vi "UHR-Fleezers Control (host) - 12.7d.vi"() -> ()   [LabVIEW 2012] (continued)
                    }
                  }
                  n1699 = local read "BD 2 Frequency 1 (MHz)"() -> (w2497:dbl)
                  n1700 = Select(t=w2498, s="Scan axis 2", f=w2497) -> (s? t:f=w2501:dbl)
                  n1701 = Add(x=w2489, y=w2501) -> (x+y=w2495:dbl)
                  n1702 = Select(t=w2495, s="Scan axis 2", f=w2498) -> (s? t:f=w2504:dbl)
                  n1703 = Select(t=w2497, s="Scan axis 2", f=w2495) -> (s? t:f=w2503:dbl)
                  n1704 = local read "BD 2 Frequency 2 (MHz)"() -> (w2506:dbl)
                  n1705 = local read "BD 2 Frequency 3 (MHz)"() -> (w2505:dbl)
                  n1706 = local read "Y RF Frequency Limits (MHz)"() -> (w2499:T16)
                  n1707 = local read "X RF Frequency Limits (MHz)"() -> (w2500:T16)
                  n1708 = local read "BD 1 Frequency 3 (MHz)"() -> (w2507:dbl)
                  n1709 = call "set RF board frequency - interlace.vi"("Board 2 Frequency Limits"=w2499, "Board 1 Frequency Limits"=w2500, "FPGA VI Reference In"=w2487, "Board 2 Frequency 3 (MHz)"=w2505, "Board 1 Frequency 3 (MHz)"=w2507, "Board 2 Frequency 2 (MHz)"=w2506, "Board 2 Frequency 1 (MHz)"=w2503, "Board 1 Frequency 2 (MHz)"=w2490, "Board 1 Frequency 1  (MHz)"=w2504) -> ()  [unwired: 1 in, 2 out]
                }
                frame #1 {
                  n1710 = And(x=w2558, y=w2555) -> (x .and. y?=w2557:bool)
                  n1711 = case "Only if were fishing and now formed tether" shown="True" w2557 {
                    tunnel: w2556 -> [w2560 w2575]
                    tunnel: [w2559 w2574] -> w2554
                    tunnel: w2553 -> [_ w2570]
                    frame False {
                      n1712 = local read "Fish for Tether"() -> (w2559:bool)
                      n1713 = case shown="False" w2559 {
                        tunnel: w2560 -> [w2561 _]
                        frame False {
                          n1714 = property on="BD 1 Frequency 1 (MHz)" class="DigNum (strict)"("Val(Sgnl)"=w2561) -> ()  [unwired: 2 in, 2 out]
                        }
                        frame True {
                        }
                      }
                    }
                    frame True {
                      w2574 = FALSE ("Fish for Tether")
                      n1715 = call <vilib>:"Beep.vi"() -> ()  [unwired: 3 in, 9 out]
                      n1716 = Number To Decimal String(number=w2570, width (-)=i16 1) -> (decimal integer string=w2568:string)
                      n1717 = Concatenate Strings("Formed tether in ", w2568, " attempt(s)." ("string")) -> (w2565:string)
                      n1718 = local read "Messages"() -> (w2572:string)
                      n1719 = local write "Fish for Tether"(w2574) -> ()
                      n1720 = call "Update messages.vi"("Message to add"=w2565, "Old message string"=w2572) -> ("New message string"=w2571:string)
                      n1721 = local write "Messages"(w2571) -> ()
                      n1722 = Get Date/Time In Seconds() -> (seconds since 1Jan1904=→"Time tether formed":timestamp)
                      n1723 = local read "Flow ON during cal?"() -> (w2562:bool)
                      n1724 = property on="Sample Channel\nFlow" class="Bool (strict)"("Val(Sgnl)"=w2562) -> (error out=w2563:errorcluster)  [unwired: 2 in, 1 out]
                      n1725 = case shown="\"2\", \"3\", \"4\", \"5\", \"6\"" "Then..." {
                        selector: "Then..." -> [_ w2578]
                        tunnel: w2575 -> [w2577 _]
                        tunnel: w2563 -> [_ _]
                        frame "1", Default {
                          n1726 = property on="BD 1 Frequency 1 (MHz)" class="DigNum (strict)"("Val(Sgnl)"=w2577) -> ()  [unwired: 2 in, 2 out]
                        }
                        frame "2", "3", "4", "5", "6" {
                          n1727 = flat-sequence {
                            tunnel: w2578 -> [w2580]
                            frame #0 {
                              n1728 = property on="Trap Delta (MHz)" class="DigNum (strict)"("Val(Sgnl)"="Move to Delta 1 (MHz)") -> ()  [unwired: 2 in, 2 out]
                            }
                            frame #1 {
                              n1729 = case shown="\"5\", \"6\"" w2580 {
                                selector: w2580 -> [w2583 w2593 _]
                                frame "3", "4" {
                                n1730 = flat-sequence {
                                tunnel: w2583 -> [w2584]
                                tunnel: [w2584] -> w2581
                                tunnel: [w2586] -> w2582
                                tunnel: w2581 -> [w2586]
                                tunnel: w2582 -> [w2590]
                                frame #0 {
                                n1731 = property on="Green Laser ON" class="Bool (strict)"("Val(Sgnl)"=TRUE ("Value (Signaling)")) -> ()  [unwired: 2 in, 2 out]
                                }
                                frame #1 {
                                n1732 = Multiply(x="Wait Before Save (s)", y=u32 1000 ("x")) -> (x*y=w2588:u32)
                                n1733 = Wait (ms)(milliseconds to wait=w2588) -> ()  [unwired: 1 out]
                                }
                                frame #2 {
                                n1734 = property on="Start Saving" class="Bool (strict)"("Value"=TRUE ("Start Saving")) -> ()  [unwired: 2 in, 2 out]
                                n1735 = case shown="\"4\"" w2590 {
                                frame Default {
                                }
                                frame "4" {
                                n1736 = property on="Fl. Triggered..." class="Bool (strict)"("Val(Sgnl)"=TRUE ("Value (Signaling)")) -> ()  [unwired: 2 in, 2 out]
                                }
                                }
                                }
                                }
                                }
                                frame "5", "6" {
                                n1737 = stacked-sequence {
                                tunnel: w2593 -> [_ _ _ _ _ _ w2605]
                                frame #0 {
                                n1738 = Replace Array Subset(array=u32[] [0] ("Index Values"), new element="Raster Set Upon Tether", index=0) -> (w2594:u32[])
                                n1739 = property on="Saved AOD Raster Scan Parameter Sets" class="Arr (strict)"("Index Values"=w2594) -> ()  [unwired: 2 in, 2 out]
                                }
                                frame #1 {
                                n1740 = Wait (ms)(milliseconds to wait=u32 500) -> ()  [unwired: 1 out]
                                }
                                frame #2 {
                                n1741 = property on="Load parameters" class="Bool (strict)"("Val(Sgnl)"=TRUE ("Value (Signaling)")) -> ()  [unwired: 2 in, 2 out]
                                n1742 = case shown="True" "Green ON During Raster" {
                                frame False {
                                }
                                frame True {
                                n1743 = property on="Green Laser ON" class="Bool (strict)"("Val(Sgnl)"=TRUE ("Value (Signaling)")) -> ()  [unwired: 2 in, 2 out]
                                }
                                }
                                }
                                frame #3 {
                                n1744 = Wait (ms)(milliseconds to wait=u32 500) -> ()  [unwired: 1 out]
                                }
                                frame #4 {
                                n1745 = property on="Trap Raster Scan" class="Bool (strict)"("Val(Sgnl)"=TRUE ("Value (Signaling)")) -> ()  [unwired: 2 in, 2 out]
                                }
                                frame #5 {
                                n1746 = Wait (ms)(milliseconds to wait=u32 2000) -> ()  [unwired: 1 out]
                                }
                                frame #6 {
                                n1747 = flat-sequence {
                                tunnel: w2605 -> [w2612]
                                frame #0 {
                                n1748 = while {
                                stop <- w2608 stop-if-true
                                n1749 = local read "Raster Scanning..."() -> (w2607:bool)
                                n1750 = local read "Saving..."() -> (w2610:bool)
                                n1751 = Wait (ms)(milliseconds to wait=u32 100) -> ()  [unwired: 1 out]
                                n1752 = Not(x=w2610) -> (.not. x?=w2609:bool)
                                n1753 = Not(x=w2607) -> (.not. x?=w2606:bool)
                                n1754 = And(x=w2609, y=w2606) -> (x .and. y?=w2608:bool)
                                }
                                }
                                frame #1 {
                                n1755 = local read "Tether"() -> (w2613:bool)
                                n1756 = case shown="True" w2613 {
                                tunnel: w2612 -> [_ w2615]
                                frame False {
                                n1757 = property on="Fish for Tether" class="Bool (strict)"("Val(Sgnl)"="Fish again after \nraster break?") -> ()  [unwired: 2 in, 2 out]
                                }
                                frame True {
                                n1758 = stacked-sequence {
                                tunnel: w2615 -> [_ w2619 _ _]
                                frame #0 {
                                n1759 = property on="Trap Delta (MHz)" class="DigNum (strict)"("Val(Sgnl)"="Move to Delta 2 (MHz)") -> ()  [unwired: 2 in, 2 out]
                                n1760 = case shown="True" "Flow ON after\ntether testing?" {
                                frame False {
                                }
                                frame True {
                                n1761 = property on="Sample Channel\nFlow" class="Bool (strict)"("Val(Sgnl)"=TRUE ("Value (Signaling)")) -> ()  [unwired: 2 in, 2 out]
                                }
                                }
                                }
                                frame #1 {
                                n1762 = flat-sequence {
                                tunnel: w2619 -> [w2621]
                                frame #0 {
                                n1763 = Wait (ms)(milliseconds to wait=u32 500) -> ()  [unwired: 1 out]
                                }
                                frame #1 {
                                n1764 = case shown="\"6\"" w2621 {
                                frame Default {
                                }
                                frame "6" {
                                n1765 = property on="Green Laser ON" class="Bool (strict)"("Val(Sgnl)"=TRUE ("Green Laser ON/Interlacing")) -> ()  [unwired: 2 in, 2 out]
                                }
                                }
                                }
                                frame #2 {
                                n1766 = Wait (ms)(milliseconds to wait=u32 500) -> ()  [unwired: 1 out]
                                }
                                frame #3 {
                                n1767 = local write "Start Saving"("Save at end (5, 6)") -> ()
                                }
                                }
                                }
                                frame #2 {
                                n1768 = local read "Bead Sep. Int. Time (s)"() -> (w2627:dbl)
                                n1769 = Multiply(x=w2627, y=1000.0) -> (x*y=w2626:dbl)
                                n1770 = Wait (ms)(milliseconds to wait=w2626) -> ()  [unwired: 1 out]
                                }
                                frame #3 {
                                n1771 = property on="Remove Offset" class="Bool (strict)"("Val(Sgnl)"=TRUE ("Value (Signaling)")) -> ()  [unwired: 2 in, 2 out]
                                }
                                }
                                }
                                }
                                }
                                }
                                }
                                }
                                }
                                frame "2", Default {
                                }
                              }
                            }
                          }
                        }
                      }
                      "Tether" <- "Tether Alarm?"
                    }
                  }
                }
                frame #2 {
                  n1772 = local read "Oscillate Set 1"() -> (w2634:bool)
                  n1773 = local read "Stop All"() -> (w2632:bool)
                  n1774 = Or(x=w2634, y=w2629) -> (x .or. y?=w2631:bool)
                  n1775 = Not(x=w2631) -> (.not. x?=w2633:bool)
                  n1776 = Compound Arithmetic op=OR(w2632, w2633) -> (w2630:bool)
                }
              }
              n1777 = node-c288() -> ()  [unwired: 2 out]
            }
            n1778 = node-c288(w2466) -> ()  [unwired: 1 out]
          }
        }
      }
      event "Fl. Triggered...": Value Change {
        n1779 = event-data() -> ()  [unwired: 7 out]
        n1780 = case shown="True" "Fl. Triggered..." {
          frame False {
          }
          frame True {
            n1781 = node-c288() -> (w2645:T23)  [unwired: 4 out]
            n1782 = timed-loop {
              timing: w2645 -> [_]
              timing-out: [_] -> w2644
              tunnel: "Action" -> [w2653]
              shift-right: [w2650] -> _
              shift-left: u8 255 -> [w2652]
              shift-right: [w2647] -> _
              shift-left: 255 -> [w2649]
              stop <- w2646 stop-if-true
              # "Reset confocal spot"
              n1783 = node-c288() -> ()  [unwired: 2 out]
              n1784 = flat-sequence {
                tunnel: w2653 -> [w2673]
                tunnel: w2652 -> [w2672]
                tunnel: [w2671] -> w2651
                tunnel: w2649 -> [w2658]
                tunnel: [w2657] -> w2648
                tunnel: [w3052] -> w2646
                tunnel: w2651 -> [w3051]
                tunnel: [w3051] -> w2650
                tunnel: [w3050] -> w2647
                tunnel: w2648 -> [w3050]
                frame #0 {
                  n1785 = local read "Delta Fl. 2"() -> (w2670:dbl)
                  n1786 = local read "Delta Fl. 1"() -> (w2665:dbl)
                  n1787 = Multiply(x="Fl. Delta Thresh. (kHz)", y=1000.0) -> (x*y=w2660:dbl)
                  n1788 = Select(t=w2665, s="APD to Watch", f=w2670) -> (s? t:f=w2661:dbl)
                  n1789 = Greater?(x=w2661, y=w2660) -> (0:w2666:bool)
                  n1790 = Or(x="Force Yank", y=w2666) -> (x .or. y?=w2664:bool)
                  n1791 = And(x=w2664, y="Yank when?") -> (x .and. y?=w2662:bool)
                  n1792 = case shown="False" w2662 {
                    tunnel: w2673 -> [w2676 w2877]
                    tunnel: w2672 -> [w2678 w2873]
                    tunnel: [w2678 w2871] -> w2671
                    tunnel: w2661 -> [w2684 _]
                    tunnel: w2660 -> [w2683 _]
                    tunnel: "Force Yank" -> [w2681 _]
                    tunnel: w2658 -> [w2680 w2870]
                    tunnel: [w2679 w2870] -> w2657
                    frame False {
                      n1793 = Negate(x=w2683) -> (-x=w2675:dbl)
                      n1794 = local write "Fl. High"(TRUE ("Fl. High")) -> ()
                      n1795 = Less?(x=w2684, y=w2675) -> (x < y?=w2682:bool)
                      n1796 = Or(x=w2681, y=w2682) -> (x .or. y?=w2677:bool)
                      n1797 = case shown="True" w2677 {
                        tunnel: w2680 -> [w2685 w2695]
                        tunnel: [w2685 w2694] -> w2679
                        tunnel: w2676 -> [_ w2693]
                        frame False {
                        }
                        frame True {
                          n1798 = flat-sequence {
                            tunnel: w2695 -> [w2701]
                            tunnel: w2693 -> [w2698]
                            tunnel: [w2700] -> w2692
                            tunnel: [w2699] -> w2691
                            tunnel: [w2698] -> w2690
                            tunnel: w2689 -> [w2697]
                            tunnel: [w2697] -> w2688
                            tunnel: w2687 -> [w2696]
                            tunnel: [w2696] -> w2686
                            tunnel: [w2772] -> w2694
                            tunnel: w2692 -> [w2772]
                            tunnel: w2691 -> [w2771]
                            tunnel: w2690 -> [w2770]
                            tunnel: w2688 -> [w2769]
                            tunnel: w2686 -> [w2768]
                            frame #0 {
                              n1799 = call <vilib>:"Beep.vi"() -> ()  [unwired: 12 in]
                              n1800 = local write "Waiting"(FALSE ("Waiting")) -> ()
                              n1801 = Increment(x=w2701) -> (x+1=w2700:i32)
                              n1802 = case shown="\"Image\"" w2698 {
                                tunnel: w2700 -> [_ w2706 _]
                                frame "Alarm", Default {
                                }
                                frame "Yank" {
                                n1803 = flat-sequence {
                                tunnel: w2706 -> [w2709]
                                tunnel: [w2708] -> w2705
                                tunnel: [w2707] -> w2704
                                tunnel: w2705 -> [w2719]
                                tunnel: w2704 -> [w2720]
                                frame #0 {
                                n1804 = local read "Yank Delay (s)"() -> (w2712:dbl)
                                n1805 = local read "N Array El"() -> (w2707:u8)
                                n1806 = Quotient & Remainder(x=w2709, y=w2707) -> (x-y*floor(x/y)=w2708:i32)  [unwired: 1 out]
                                n1807 = Multiply(x=w2712, y=1000.0) -> (x*y=w2710:dbl)
                                n1808 = Wait (ms)(milliseconds to wait=w2710) -> ()  [unwired: 1 out]
                                }
                                frame #1 {
                                n1809 = local read "Yank to which?"() -> (w2714:bool)
                                n1810 = local read "Random Choice"() -> (w2724:bool)
                                n1811 = local read "Yank to Trap Delta (MHz)"() -> (w2717:dbl[])
                                n1812 = local read "Yank to SP"() -> (w2718:dbl[])
                                n1813 = Random Number (0-1)() -> (number: 0 to 1=w2723:dbl)
                                n1814 = Multiply(x=w2720, y=w2723) -> (x*y=w2722:dbl)
                                n1815 = Round Toward -Infinity(1:w2722) -> (0:w2721:dbl)
                                n1816 = Select(t=w2721, s=w2724, f=w2719) -> (s? t:f=w2715:dbl)
                                n1817 = Select(t=w2717, s=w2714, f=w2718) -> (s? t:f=w2716:dbl[])
                                n1818 = Index Array(array=w2716, index=w2715) -> (element=w2713:dbl)
                                n1819 = case shown="True" w2714 {
                                tunnel: w2713 -> [w2725 w2752]
                                frame False {
                                n1820 = flat-sequence {
                                tunnel: w2725 -> [w2726]
                                frame #0 {
                                n1821 = property on="Trap Pos FB SP" class="DigNum (strict)"("Val(Sgnl)"=w2726) -> ()  [unwired: 2 in, 2 out]
                                }
                                frame #1 {
                                n1822 = Wait (ms)(milliseconds to wait=u32 700) -> ()  [unwired: 1 out]
                                }
                                frame #2 {
                                n1823 = local read "Action (%)"() -> (w2731:dbl)
                                n1824 = Absolute Value(x=w2731) -> (abs(x)=w2730:dbl)
                                n1825 = Greater?(x=w2730, y=70.0) -> (0:w2728:bool)
                                n1826 = property on="Remove Action Offset" class="Bool (strict)"("Val(Sgnl)"=w2728) -> ()  [unwired: 2 in, 2 out]
                                }
                                frame #3 {
                                n1827 = for {
                                N: 4 -> [_]
                                n1828 = flat-sequence {
                                frame #0 {
                                n1829 = Wait (ms)(milliseconds to wait=u32 500) -> ()  [unwired: 1 out]
                                }
                                frame #1 {
                                n1830 = local read "Action (%)"() -> (w2737:dbl)
                                n1831 = Absolute Value(x=w2737) -> (abs(x)=w2736:dbl)
                                n1832 = Greater?(x=w2736, y=70.0) -> (0:w2734:bool)
                                n1833 = property on="Remove Action Offset" class="Bool (strict)"("Val(Sgnl)"=w2734) -> ()  [unwired: 2 in, 2 out]
                                }
                                }
                                }
                                }
                                frame #4 {
                                n1834 = Wait (ms)(milliseconds to wait=u32 500) -> ()  [unwired: 1 out]
                                }
                                frame #5 {
                                n1835 = local read "Mean"() -> (w2745:dbl)
                                n1836 = Greater?(x=w2745, y=11.0) -> (0:w2739:bool)
                                n1837 = Not(x=w2739) -> (.not. x?=w2740:bool)
                                n1838 = And(x=w2740, y="Shift confocal") -> (x .and. y?=w2742:bool)
                                n1839 = And(x=w2739, y="Shift confocal") -> (x .and. y?=w2743:bool)
                                n1840 = case shown="True" w2743 {
                                frame False {
                                }
                                frame True {
                                n1841 = local read "Confocal Y 2 (V)"() -> (w2749:dbl)
                                n1842 = local read "Confocal X 2 (V)"() -> (w2748:dbl)
                                n1843 = property on="AO1" class="Slide (strict)"("Val(Sgnl)"=w2749) -> ()  [unwired: 2 in, 2 out]
                                n1844 = property on="AO2" class="Slide (strict)"("Val(Sgnl)"=w2748) -> ()  [unwired: 2 in, 2 out]
                                }
                                }
                                n1845 = case shown="True" w2742 {
                                frame False {
                                }
                                frame True {
                                n1846 = local read "Confocal Y 1 (V)"() -> (w2747:dbl)
                                n1847 = local read "Confocal X 1 (V)"() -> (w2746:dbl)
                                n1848 = property on="AO1" class="Slide (strict)"("Val(Sgnl)"=w2747) -> ()  [unwired: 2 in, 2 out]
                                n1849 = property on="AO2" class="Slide (strict)"("Val(Sgnl)"=w2746) -> ()  [unwired: 2 in, 2 out]
                                }
                                }
                                }
                                frame #6 {
                                n1850 = Wait (ms)(milliseconds to wait=u32 1500) -> ()  [unwired: 1 out]
                                }
                                frame #7 {
                                n1851 = property on="Rem fb disp offset" class="Bool (strict)"("Val(Sgnl)"=TRUE ("Value (Signaling)")) -> ()  [unwired: 2 in, 2 out]
                                }
                                }
                                }
                                frame True {
                                n1852 = flat-sequence {
                                tunnel: w2752 -> [w2753]
                                frame #0 {
                                n1853 = property on="Trap Delta (MHz)" class="DigNum (strict)"("Val(Sgnl)"=w2753) -> ()  [unwired: 2 in, 2 out]
                                }
                                frame #1 {
                                n1854 = Wait (ms)(milliseconds to wait=u32 500) -> ()  [unwired: 1 out]
                                }
                                frame #2 {
                                n1855 = local read "Shift confocal"() -> (w2759:bool)
                                n1856 = local read "Mean"() -> (w2761:dbl)
                                n1857 = Greater?(x=w2761, y=11.0) -> (0:w2758:bool)
                                n1858 = Not(x=w2758) -> (.not. x?=w2757:bool)
                                n1859 = And(x=w2757, y=w2759) -> (x .and. y?=w2755:bool)
                                n1860 = And(x=w2758, y=w2759) -> (x .and. y?=w2756:bool)
                                n1861 = case shown="True" w2756 {
                                frame False {
                                }
                                frame True {
                                n1862 = local read "Confocal Y 2 (V)"() -> (w2765:dbl)
                                n1863 = local read "Confocal X 2 (V)"() -> (w2764:dbl)
                                n1864 = property on="AO2" class="Slide (strict)"("Val(Sgnl)"=w2764) -> ()  [unwired: 2 in, 2 out]
                                n1865 = property on="AO1" class="Slide (strict)"("Val(Sgnl)"=w2765) -> ()  [unwired: 2 in, 2 out]
                                }
                                }
                                n1866 = case shown="True" w2755 {
                                frame False {
                                }
                                frame True {
                                n1867 = local read "Confocal X 1 (V)"() -> (w2762:dbl)
                                n1868 = local read "Confocal Y 1 (V)"() -> (w2763:dbl)
                                n1869 = property on="AO2" class="Slide (strict)"("Val(Sgnl)"=w2762) -> ()  [unwired: 2 in, 2 out]
                                n1870 = property on="AO1" class="Slide (strict)"("Val(Sgnl)"=w2763) -> ()  [unwired: 2 in, 2 out]
                                }
                                }
                                }
                                }
                                }
                                }
                                }
                                }
                                }
                                frame "Image" {
                                n1871 = property on="Confocal Image" class="Bool (strict)"("Val(Sgnl)"=TRUE ("Value (Signaling)")) -> ()  [unwired: 2 in, 2 out]
                                }
                              }
                              n1872 = local write "Fl. High"(FALSE ("Fl. High")) -> ()
                              n1873 = local read "Time (s)"() -> (w2699:dbl)
                            }
                            frame #1 {
                              n1874 = case shown="True" "Auto F Reset" {
                                tunnel: w2771 -> [_ w2776]
                                tunnel: w2770 -> [_ w2775]
                                tunnel: w2769 -> [_ w2774]
                                tunnel: w2768 -> [_ w2773]
                                frame False {
                                }
                                frame True {
                                n1875 = node-c288() -> (w2778:T23)  [unwired: 4 in]
                                n1876 = timed-loop {
                                timing: w2778 -> [_]
                                timing-out: [_] -> w2777
                                tunnel: w2776 -> [w2783]
                                tunnel: w2775 -> [w2782]
                                tunnel: w2774 -> [w2781]
                                tunnel: w2773 -> [w2780]
                                stop <- w2779 stop-if-true
                                n1877 = node-c288() -> ()  [unwired: 1 in, 1 out]
                                n1878 = local read "Fl. Delta Thresh. (kHz)"() -> (w2792:dbl)
                                n1879 = local read "APD to Watch"() -> (w2793:bool)
                                n1880 = local read "Delta Fl. 1"() -> (w2794:dbl)
                                n1881 = local read "Delta Fl. 2"() -> (w2795:dbl)
                                n1882 = local read "Fl. Triggered..."() -> (w2786:bool)
                                n1883 = local read "Stop All"() -> (w2787:bool)
                                n1884 = local read "Reset Force"() -> (w2785:bool)
                                n1885 = Multiply(x=w2792, y=1000.0) -> (x*y=w2790:dbl)
                                n1886 = Select(t=w2794, s=w2793, f=w2795) -> (s? t:f=w2789:dbl)
                                n1887 = Not(x=w2786) -> (.not. x?=w2784:bool)
                                n1888 = Greater?(x=w2789, y=w2790) -> (0:w2788:bool)
                                n1889 = Compound Arithmetic op=OR(w2788, w2787, w2784, w2785) -> (w2779:bool)
                                n1890 = case shown="True" w2779 {
                                tunnel: w2783 -> [_ w2799]
                                tunnel: w2782 -> [_ w2803]
                                tunnel: w2781 -> [_ w2802]
                                tunnel: w2780 -> [_ w2801]
                                frame False {
                                }
                                frame True {
                                n1891 = case shown="\"Yank\"" w2803 {
                                tunnel: w2802 -> [_ w2813]
                                tunnel: w2801 -> [_ w2811]
                                frame "Image", Default {
                                }
                                frame "Yank" {
                                n1892 = flat-sequence {
                                tunnel: [w2816] -> w2814
                                tunnel: w2813 -> [w2816]
                                tunnel: [w2815] -> w2812
                                tunnel: w2811 -> [w2815]
                                tunnel: w2814 -> [w2822]
                                tunnel: w2812 -> [w2820]
                                frame #0 {
                                n1893 = local read "Yank Delay (s)"() -> (w2819:dbl)
                                n1894 = Multiply(x=w2819, y=1000.0) -> (x*y=w2817:dbl)
                                n1895 = Wait (ms)(milliseconds to wait=w2817) -> ()  [unwired: 1 out]
                                }
                                frame #1 {
                                n1896 = local read "Yank to which?"() -> (w2821:bool)
                                n1897 = case shown="False" w2821 {
                                tunnel: w2822 -> [_ w2850]
                                tunnel: w2820 -> [w2823 _]
                                frame False {
                                n1898 = flat-sequence {
                                tunnel: w2823 -> [w2824]
                                frame #0 {
                                n1899 = property on="Trap Pos FB SP" class="DigNum (strict)"("Val(Sgnl)"=w2824) -> ()  [unwired: 2 in, 2 out]
                                }
                                frame #1 {
                                n1900 = Wait (ms)(milliseconds to wait=u32 700) -> ()  [unwired: 1 out]
                                }
                                frame #2 {
                                n1901 = local read "Action (%)"() -> (w2829:dbl)
                                n1902 = Absolute Value(x=w2829) -> (abs(x)=w2828:dbl)
                                n1903 = Greater?(x=w2828, y=70.0) -> (0:w2826:bool)
                                n1904 = property on="Remove Action Offset" class="Bool (strict)"("Val(Sgnl)"=w2826) -> ()  [unwired: 2 in, 2 out]
                                }
                                frame #3 {
                                n1905 = for {
                                N: 4 -> [_]
                                n1906 = flat-sequence {
                                frame #0 {
                                n1907 = Wait (ms)(milliseconds to wait=u32 500) -> ()  [unwired: 1 out]
                                }
                                frame #1 {
                                n1908 = local read "Action (%)"() -> (w2835:dbl)
                                n1909 = Absolute Value(x=w2835) -> (abs(x)=w2834:dbl)
                                n1910 = Greater?(x=w2834, y=70.0) -> (0:w2832:bool)
                                n1911 = property on="Remove Action Offset" class="Bool (strict)"("Val(Sgnl)"=w2832) -> ()  [unwired: 2 in, 2 out]
                                }
                                }
                                }
                                }
                                frame #4 {
                                n1912 = Wait (ms)(milliseconds to wait=u32 500) -> ()  [unwired: 1 out]
                                }
                                frame #5 {
                                n1913 = local read "Shift confocal"() -> (w2840:bool)
                                n1914 = local read "Mean"() -> (w2843:dbl)
                                n1915 = Greater?(x=w2843, y=11.0) -> (0:w2839:bool)
                                n1916 = Not(x=w2839) -> (.not. x?=w2838:bool)
                                n1917 = And(x=w2839, y=w2840) -> (x .and. y?=w2841:bool)
                                n1918 = And(x=w2838, y=w2840) -> (x .and. y?=w2837:bool)
                                n1919 = case shown="True" w2841 {
                                frame False {
                                }
                                frame True {
                                n1920 = local read "Confocal X 2 (V)"() -> (w2846:dbl)
                                n1921 = local read "Confocal Y 2 (V)"() -> (w2847:dbl)
                                n1922 = property on="AO2" class="Slide (strict)"("Val(Sgnl)"=w2846) -> ()  [unwired: 2 in, 2 out]
                                n1923 = property on="AO1" class="Slide (strict)"("Val(Sgnl)"=w2847) -> ()  [unwired: 2 in, 2 out]
                                }
                                }
                                n1924 = case shown="True" w2837 {
                                frame False {
                                }
                                frame True {
                                n1925 = local read "Confocal Y 1 (V)"() -> (w2845:dbl)
                                n1926 = local read "Confocal X 1 (V)"() -> (w2844:dbl)
                                n1927 = property on="AO1" class="Slide (strict)"("Val(Sgnl)"=w2845) -> ()  [unwired: 2 in, 2 out]
                                n1928 = property on="AO2" class="Slide (strict)"("Val(Sgnl)"=w2844) -> ()  [unwired: 2 in, 2 out]
                                }
                                }
                                }
                                frame #6 {
                                n1929 = Wait (ms)(milliseconds to wait=u32 1500) -> ()  [unwired: 1 out]
                                }
                                frame #7 {
                                n1930 = property on="Rem fb disp offset" class="Bool (strict)"("Val(Sgnl)"=TRUE ("Value (Signaling)")) -> ()  [unwired: 2 in, 2 out]
                                }
                                }
                                }
                                frame True {
                                n1931 = flat-sequence {
                                tunnel: w2850 -> [w2851]
                                frame #0 {
                                n1932 = property on="Trap Delta (MHz)" class="DigNum (strict)"("Val(Sgnl)"=w2851) -> ()  [unwired: 2 in, 2 out]
                                }
                                frame #1 {
                                n1933 = Wait (ms)(milliseconds to wait=u32 500) -> ()  [unwired: 1 out]
                                }
                                frame #2 {
                                n1934 = local read "Shift confocal"() -> (w2857:bool)
                                n1935 = local read "Mean"() -> (w2858:dbl)
                                n1936 = Greater?(x=w2858, y=11.0) -> (0:w2856:bool)
                                n1937 = And(x=w2856, y=w2857) -> (x .and. y?=w2854:bool)
                                n1938 = Not(x=w2856) -> (.not. x?=w2855:bool)
                                n1939 = And(x=w2855, y=w2857) -> (x .and. y?=w2853:bool)
                                n1940 = case shown="True" w2854 {
                                frame False {
                                }
                                frame True {
                                n1941 = local read "Confocal Y 2 (V)"() -> (w2863:dbl)
                                n1942 = local read "Confocal X 2 (V)"() -> (w2862:dbl)
                                n1943 = property on="AO1" class="Slide (strict)"("Val(Sgnl)"=w2863) -> ()  [unwired: 2 in, 2 out]
                                n1944 = property on="AO2" class="Slide (strict)"("Val(Sgnl)"=w2862) -> ()  [unwired: 2 in, 2 out]
                                }
                                }
                                n1945 = case shown="True" w2853 {
                                frame False {
                                }
                                frame True {
                                n1946 = local read "Confocal Y 1 (V)"() -> (w2861:dbl)
                                n1947 = local read "Confocal X 1 (V)"() -> (w2860:dbl)
                                n1948 = property on="AO2" class="Slide (strict)"("Val(Sgnl)"=w2860) -> ()  [unwired: 2 in, 2 out]
                                n1949 = property on="AO1" class="Slide (strict)"("Val(Sgnl)"=w2861) -> ()  [unwired: 2 in, 2 out]
                                }
                                }
                                }
                                }
                                }
                                }
                                }
                                }
                                }
                                }
                                n1950 = local read "Time (s)"() -> (w2798:dbl)
                                n1951 = Subtract(x=w2799, y=w2798) -> (x-y=w2810:dbl)
                                n1952 = Number To Decimal String(number=w2810, width (-)=i16 0) -> (decimal integer string=w2808:string)
                                n1953 = Concatenate Strings(w2808, " s fluorescence event") -> (w2805:string)
                                n1954 = local read "Messages"() -> (w2806:string)
                                n1955 = local write "Duration (s)"(w2810) -> ()
                                n1956 = call "Update messages.vi"("Message to add"=w2805, "Old message string"=w2806) -> ("New message string"=w2804:string)
                                n1957 = local write "Messages"(w2804) -> ()
                                n1958 = call <vilib>:"Beep.vi"() -> ()  [unwired: 12 in]
                                n1959 = local write "Reset Force"(FALSE ("Force Reset")) -> ()
                                n1960 = local write "Fl. High"(TRUE ("Fl. High")) -> ()
                                n1961 = local write "Waiting"(TRUE ("Waiting")) -> ()
                                }
                                }
                                n1962 = node-c288() -> ()  [unwired: 1 in, 1 out]
                                }
                                n1963 = node-c288(w2777) -> ()  [unwired: 1 out]
                                }
                              }
                            }
                          }
                          n1964 = local read "Trap Delta (MHz)"() -> (w2689:dbl)
                          n1965 = local read "Trap Pos FB SP"() -> (w2687:fxp<+/-,16,1>)
                        }
                      }
                    }
                    frame True {
                      n1966 = flat-sequence {
                        tunnel: w2874 -> [w2884]
                        tunnel: [w2884] -> w2878
                        tunnel: w2877 -> [w2883]
                        tunnel: [w2883] -> w2876
                        tunnel: [w2882] -> w2875
                        tunnel: w2873 -> [w2881]
                        tunnel: [w2880] -> w2872
                        tunnel: w2869 -> [w2879]
                        tunnel: [w2879] -> w2868
                        tunnel: w2878 -> [w2954]
                        tunnel: w2876 -> [w2953]
                        tunnel: w2875 -> [w2952]
                        tunnel: w2872 -> [w2951]
                        tunnel: w2868 -> [w2950]
                        tunnel: [w2951] -> w2871
                        frame #0 {
                          n1967 = call <vilib>:"Beep.vi"() -> ()  [unwired: 3 in, 9 out]
                          n1968 = local write "Waiting"(FALSE ("Waiting")) -> ()
                          n1969 = Increment(x=w2881) -> (x+1=w2880:u8)
                          n1970 = case shown="\"Yank\"" w2883 {
                            tunnel: w2880 -> [_ _ w2890]
                            frame "Image" {
                              n1971 = property on="Confocal Image" class="Bool (strict)"("Val(Sgnl)"=TRUE ("Value (Signaling)")) -> ()  [unwired: 2 in, 2 out]
                            }
                            frame "Alarm", Default {
                            }
                            frame "Yank" {
                              n1972 = flat-sequence {
                                tunnel: w2890 -> [w2893]
                                tunnel: [w2892] -> w2889
                                tunnel: ["N Array El"] -> w2888
                                tunnel: w2889 -> [w2907]
                                tunnel: w2888 -> [w2903]
                                frame #0 {
                                n1973 = Multiply(x="Yank Delay (s)", y=1000.0) -> (x*y=w2896:dbl)
                                n1974 = Quotient & Remainder(x=w2893, y="N Array El") -> (x-y*floor(x/y)=w2892:u8)  [unwired: 1 out]
                                n1975 = Wait (ms)(milliseconds to wait=w2896) -> ()  [unwired: 1 out]
                                }
                                frame #1 {
                                n1976 = Random Number (0-1)() -> (number: 0 to 1=w2904:dbl)
                                n1977 = Multiply(x=w2903, y=w2904) -> (x*y=w2902:dbl)
                                n1978 = Round Toward -Infinity(1:w2902) -> (0:w2901:dbl)
                                n1979 = Select(t=w2901, s="Random Choice", f=w2907) -> (s? t:f=w2905:dbl)
                                n1980 = Select(t="Yank to Trap Delta (MHz)", s="Yank to which?", f="Yank to SP") -> (s? t:f=w2898:dbl[])
                                n1981 = Index Array(array=w2898, index=w2905) -> (element=w2908:dbl)
                                n1982 = case shown="False" "Yank to which?" {
                                tunnel: w2908 -> [w2909 w2935]
                                frame False {
                                n1983 = flat-sequence {
                                tunnel: w2909 -> [w2910]
                                frame #0 {
                                n1984 = property on="Trap Pos FB SP" class="DigNum (strict)"("Val(Sgnl)"=w2910) -> ()  [unwired: 2 in, 2 out]
                                }
                                frame #1 {
                                n1985 = Wait (ms)(milliseconds to wait=u32 700) -> ()  [unwired: 1 out]
                                }
                                frame #2 {
                                n1986 = local read "Action (%)"() -> (w2915:dbl)
                                n1987 = Absolute Value(x=w2915) -> (abs(x)=w2914:dbl)
                                n1988 = Greater?(x=w2914, y=70.0) -> (0:w2912:bool)
                                n1989 = property on="Remove Action Offset" class="Bool (strict)"("Val(Sgnl)"=w2912) -> ()  [unwired: 2 in, 2 out]
                                }
                                frame #3 {
                                n1990 = for {
                                N: 4 -> [_]
                                n1991 = flat-sequence {
                                frame #0 {
                                n1992 = Wait (ms)(milliseconds to wait=u32 500) -> ()  [unwired: 1 out]
                                }
                                frame #1 {
                                n1993 = local read "Action (%)"() -> (w2921:dbl)
                                n1994 = Absolute Value(x=w2921) -> (abs(x)=w2920:dbl)
                                n1995 = Greater?(x=w2920, y=70.0) -> (0:w2918:bool)
                                n1996 = property on="Remove Action Offset" class="Bool (strict)"("Val(Sgnl)"=w2918) -> ()  [unwired: 2 in, 2 out]
                                }
                                }
                                }
                                }
                                frame #4 {
                                n1997 = local read "Shift confocal"() -> (w2925:bool)
                                n1998 = local read "Mean"() -> (w2928:dbl)
                                n1999 = Greater?(x=w2928, y=11.0) -> (0:w2924:bool)
                                n2000 = Not(x=w2924) -> (.not. x?=w2923:bool)
                                n2001 = And(x=w2923, y=w2925) -> (x .and. y?=w2922:bool)
                                n2002 = And(x=w2924, y=w2925) -> (x .and. y?=w2926:bool)
                                n2003 = case shown="True" w2926 {
                                frame False {
                                }
                                frame True {
                                n2004 = local read "Confocal X 2 (V)"() -> (w2931:dbl)
                                n2005 = local read "Confocal Y 2 (V)"() -> (w2932:dbl)
                                n2006 = property on="AO2" class="Slide (strict)"("Val(Sgnl)"=w2931) -> ()  [unwired: 2 in, 2 out]
                                n2007 = property on="AO1" class="Slide (strict)"("Val(Sgnl)"=w2932) -> ()  [unwired: 2 in, 2 out]
                                }
                                }
                                n2008 = case shown="True" w2922 {
                                frame False {
                                }
                                frame True {
                                n2009 = local read "Confocal X 1 (V)"() -> (w2929:dbl)
                                n2010 = local read "Confocal Y 1 (V)"() -> (w2930:dbl)
                                n2011 = property on="AO1" class="Slide (strict)"("Val(Sgnl)"=w2930) -> ()  [unwired: 2 in, 2 out]
                                n2012 = property on="AO2" class="Slide (strict)"("Val(Sgnl)"=w2929) -> ()  [unwired: 2 in, 2 out]
                                }
                                }
                                }
                                frame #5 {
                                n2013 = Wait (ms)(milliseconds to wait=u32 1500) -> ()  [unwired: 1 out]
                                }
                                frame #6 {
                                n2014 = property on="Rem fb disp offset" class="Bool (strict)"("Val(Sgnl)"=TRUE ("Value (Signaling)")) -> ()  [unwired: 2 in, 2 out]
                                }
                                }
                                }
                                frame True {
                                n2015 = flat-sequence {
                                tunnel: w2935 -> [w2936]
                                frame #0 {
                                n2016 = property on="Trap Delta (MHz)" class="DigNum (strict)"("Val(Sgnl)"=w2936) -> ()  [unwired: 2 in, 2 out]
                                }
                                frame #1 {
                                n2017 = Wait (ms)(milliseconds to wait=u32 500) -> ()  [unwired: 1 out]
                                }
                                frame #2 {
                                n2018 = local read "Shift confocal"() -> (w2940:bool)
                                n2019 = local read "Mean"() -> (w2938:dbl)
                                n2020 = Greater?(x=w2938, y=11.0) -> (0:w2941:bool)
                                n2021 = Not(x=w2941) -> (.not. x?=w2942:bool)
                                n2022 = And(x=w2942, y=w2940) -> (x .and. y?=w2944:bool)
                                n2023 = And(x=w2941, y=w2940) -> (x .and. y?=w2943:bool)
                                n2024 = case shown="True" w2943 {
                                frame False {
                                }
                                frame True {
                                n2025 = local read "Confocal Y 2 (V)"() -> (w2948:dbl)
                                n2026 = local read "Confocal X 2 (V)"() -> (w2947:dbl)
                                n2027 = property on="AO1" class="Slide (strict)"("Val(Sgnl)"=w2948) -> ()  [unwired: 2 in, 2 out]
                                n2028 = property on="AO2" class="Slide (strict)"("Val(Sgnl)"=w2947) -> ()  [unwired: 2 in, 2 out]
                                }
                                }
                                n2029 = case shown="True" w2944 {
                                frame False {
                                }
                                frame True {
                                n2030 = local read "Confocal X 1 (V)"() -> (w2945:dbl)
                                n2031 = local read "Confocal Y 1 (V)"() -> (w2946:dbl)
                                n2032 = property on="AO2" class="Slide (strict)"("Val(Sgnl)"=w2945) -> ()  [unwired: 2 in, 2 out]
                                n2033 = property on="AO1" class="Slide (strict)"("Val(Sgnl)"=w2946) -> ()  [unwired: 2 in, 2 out]
                                }
                                }
                                }
                                }
                                }
                                }
                                }
                              }
                            }
                          }
                          n2034 = local read "Time (s)"() -> (w2882:dbl)
                          "Fl. High" <- TRUE ("Yanking")
                        }
                        frame #1 {
                          n2035 = local read "Auto F Reset"() -> (w2949:bool)
                          n2036 = case shown="True" w2949 {
                            tunnel: w2954 -> [_ w2958]
                            tunnel: w2953 -> [_ w2957]
                            tunnel: w2952 -> [_ w2956]
                            tunnel: w2950 -> [_ w2955]
                            frame False {
                            }
                            frame True {
                              n2037 = node-c288() -> (w2960:T23)  [unwired: 4 out]
                              n2038 = timed-loop {
                                timing: w2960 -> [_]
                                timing-out: [_] -> w2959
                                tunnel: w2958 -> [w2978]
                                tunnel: w2957 -> [w2977]
                                tunnel: w2956 -> [w2976]
                                tunnel: w2955 -> [w2975]
                                stop <- w2961 stop-if-true
                                n2039 = node-c288() -> ()  [unwired: 2 out]
                                n2040 = local read "Fl. Delta Thresh. (kHz)"() -> (w2969:dbl)
                                n2041 = local read "Fl. Triggered..."() -> (w2974:bool)
                                n2042 = local read "Delta Fl. 1"() -> (w2965:dbl)
                                n2043 = local read "Delta Fl. 2"() -> (w2963:dbl)
                                n2044 = local read "Stop All"() -> (w2972:bool)
                                n2045 = local read "APD to Watch"() -> (w2964:bool)
                                n2046 = Select(t=w2965, s=w2964, f=w2963) -> (s? t:f=w2962:dbl)
                                n2047 = Not(x=w2974) -> (.not. x?=w2973:bool)
                                n2048 = Multiply(x=w2969, y=1000.0) -> (x*y=w2968:dbl)
                                n2049 = Negate(x=w2968) -> (-x=w2967:dbl)
                                n2050 = Less?(x=w2962, y=w2967) -> (x < y?=w2971:bool)
                                n2051 = Compound Arithmetic op=OR(w2971, w2972, w2973, "Reset Force") -> (w2961:bool)